vi "HFRR ADV v038.vi"() -> ()   [LabVIEW 2025] (continued)
                    n2637 = local write "Temperature ( Deg C )"(w3212) -> ()
                    n2638 = Number To Fractional String(number=w3190, width (-)=i16 9 ("precision (6)"), precision (6)=i16 6) -> (F-format string=w3236:string)  [unwired: 1 in]
                    n2639 = Number To Fractional String(number=w3216, width (-)=i16 9 ("precision (6)"), precision (6)=i16 3) -> (F-format string=w3235:string)  [unwired: 1 in]
                    n2640 = Number To Fractional String(number=w3212, width (-)=i16 9 ("precision (6)"), precision (6)=i16 3) -> (F-format string=w3232:string)  [unwired: 1 in]
                    n2641 = Number To Fractional String(number=w3211, width (-)=i16 9 ("precision (6)"), precision (6)=i16 3) -> (F-format string=w3229:string)  [unwired: 1 in]
                    n2642 = Number To Fractional String(number=0.0, width (-)=i16 9 ("precision (6)"), precision (6)=i16 3) -> (F-format string=w3226:string)  [unwired: 1 in]
                    n2643 = Number To Fractional String(number=w3221, width (-)=i16 9 ("precision (6)"), precision (6)=i16 3) -> (F-format string=w3222:string)  [unwired: 1 in]
                    n2644 = Number To Fractional String(number=w3218, width (-)=i16 9 ("precision (6)"), precision (6)=i16 3) -> (F-format string=w3217:string)  [unwired: 1 in]
                    n2645 = Number To Fractional String(number=w3209, width (-)=i16 9 ("precision (6)"), precision (6)=i16 6) -> (F-format string=w3244:string)  [unwired: 1 in]
                    n2646 = Number To Fractional String(number=w3243, width (-)=i16 14 ("precision (6)"), precision (6)=i16 3) -> (F-format string=w3245:string)  [unwired: 1 in]
                    n2647 = Bundle("y"=1.02, "LVDT STROKE DISPLAY"=w3190, "y"=0.98) -> (w3210:T31)  [unwired: 1 in]
                    n2648 = Number To Fractional String(number="Ambient Humidity :", width (-)=i16 9 ("precision (6)"), precision (6)=i16 6) -> (F-format string=w3202:string)  [unwired: 1 in]
                    n2649 = local read "RUN"() -> (w3208:bool)
                    n2650 = case shown="True" w3208 {
                      tunnel: w3210 -> [_ w3261]
                      tunnel: w3190 -> [_ w3260]
                      tunnel: w3190 -> [_ w3258]
                      tunnel: w3190 -> [_ w3259]
                      frame False {
                      }
                      frame True {
                        "Stroke ( mm )" <- w3261
                        "Stroke ( mm )" <- w3261
                        "Stroke 4" <- w3260
                        "Stroke 3" <- w3258
                        "Stroke 2" <- w3259
                        "measured_stroke" <- w3258
                      }
                    }
                    n2651 = Concatenate Strings(w3245, w3204, w3244, w3204, w3236, w3204, w3235, w3204, w3232, w3204, w3229, w3204, w3226, w3204, w3222, w3204, w3217, w3204, w3202, "\r") -> (w3242:string)
                    n2652 = call <vilib>:"Write Characters To File.vi"("append to file? (new file:F)"=TRUE, "character string"=w3242, "file path (dialog if empty)"=w3195) -> ()  [unwired: 2 in, 1 out]
                    "refresh flag" <- TRUE ("refresh flag")
                    "LVDT STROKE Actual" <- w3188
                  }
                }
                n2653 = case shown="True" w3110 {
                  tunnel: w3120 -> [_ w3146]
                  tunnel: w3125 -> [_ w3156]
                  tunnel: [0.0 w3152] -> _
                  tunnel: w3119 -> [_ w3151]
                  tunnel: [0.0 w3150] -> _
                  tunnel: w3109 -> [_ w3150]
                  tunnel: w3123 -> [w3139 _]
                  frame False {
                    n2654 = local write "acq timer"(w3139) -> ()
                    n2655 = local write "Test Duration Status"(0.0 ("Test Duration Status")) -> ()
                  }
                  frame True {
                    n2656 = local read "Set Hz"() -> (w3153:dbl)
                    n2657 = local write "Elapsed time"(w3146) -> ()
                    n2658 = local read "test time"() -> (w3145:dbl)
                    n2659 = Multiply(x=w3156, y=w3153) -> (x*y=w3155:dbl)
                    n2660 = case shown="False" w3151 {
                      tunnel: w3155 -> [w3157 _]
                      tunnel: [w3157 1.0] -> w3152
                      frame False {
                        n2661 = local write "Cycles elapsed"(w3157) -> ()
                      }
                      frame True {
                      }
                    }
                    n2662 = Greater?(x=w3146, y=w3145) -> (0:w3154:bool)
                    n2663 = Subtract(x=w3145, y=w3146) -> (x-y=w3144:dbl)
                    n2664 = Multiply(x=w3144, y=60.0) -> (x*y=w3143:dbl)
                    n2665 = local write "Time Remaining"(w3143) -> ()
                    n2666 = local write "Remaining Time"(w3143) -> ()
                    n2667 = case shown="True" w3154 {
                      frame False {
                      }
                      frame True {
                        n2668 = stacked-sequence {
                          frame #0 {
                            w3162 = T19."Enabled" ("Disabled")
                            w3161 = FALSE ("TEST FILE NAM,E SAVED")
                            w3163 = "" ("FILE")
                            w3164 = TRUE ("Visible")
                            n2669 = local write "Humidity"(FALSE ("Humidity")) -> ()
                            n2670 = local write "RUN"(FALSE ("OK Button 2")) -> ()
                            n2671 = local write "Heater Button"(FALSE ("Heater Button")) -> ()
                            n2672 = local write "Auto Start Test"(FALSE ("Auto Start Test")) -> ()
                            n2673 = local write "TestCompFlg"(TRUE ("StpFlg")) -> ()
                            n2674 = local read "Humidity ( %RH )"() -> (→"Rh After":dbl)
                            n2675 = property on="STOP 2" class="Bool (strict)"("Disabled"=u8 0) -> ()  [unwired: 2 in, 2 out]
                            n2676 = local read "EVENT LOG"() -> (w3169:string)
                            n2677 = call "Event Log.vi"("Content"="Test Completed", "EVENT LOG"=w3169) -> ("EVENT LOG"=w3168:string)  [unwired: 8 in, 1 out]
                            n2678 = property on="RUN" class="Bool (strict)"("Visible"=w3164) -> ()  [unwired: 2 in, 2 out]
                            n2679 = property on="Auto Start Test" class="Bool (strict)"("Visible"=w3164) -> ()  [unwired: 2 in, 2 out]
                            n2680 = local write "Batch Ref Num :"(w3163) -> ()
                            n2681 = local write "FILE"(w3163) -> ()
                            n2682 = local write "EVENT LOG"(w3168) -> ()
                            n2683 = local write "TEST FILE NAM,E SAVED"(w3161) -> ()
                            n2684 = local write "Fuel Discription :"(w3163) -> ()
                            n2685 = local write "START TEMP"(w3161) -> ()
                            n2686 = local write "Remarks :"(w3163) -> ()
                            n2687 = local write "Main Dashboard Buttons"(T1."Imaging" ("Main Dashboard Buttons")) -> ()
                            n2688 = local write "Main Tab"(T2."Adv Scar" ("Main Tab")) -> ()
                            n2689 = property on="FRICVALZ 2" class="Bool (strict)"("DisabledEnum"=w3162) -> ()  [unwired: 2 in, 2 out]
                            n2690 = property on="FRICVALZ 3" class="Bool (strict)"("DisabledEnum"=w3162) -> ()  [unwired: 2 in, 2 out]
                            n2691 = property on="FRICVALZ 4" class="Bool (strict)"("DisabledEnum"=w3162) -> ()  [unwired: 2 in, 2 out]
                          }
                          frame #1 {
                            n2692 = Wait (ms)(milliseconds to wait=u32 1500) -> ()  [unwired: 1 out]
                          }
                          frame #2 {
                            n2693 = local write "Due Write"("VC;0") -> ()
                          }
                          frame #3 {
                            n2694 = Wait (ms)(milliseconds to wait=u32 1500) -> ()  [unwired: 1 out]
                          }
                          frame #4 {
                            n2695 = local write "Due Write"("VC;0") -> ()
                          }
                          frame #5 {
                            n2696 = Wait (ms)(milliseconds to wait=u32 1500) -> ()  [unwired: 1 out]
                          }
                          frame #6 {
                            n2697 = local write "Due Write"("ST;0") -> ()
                          }
                          frame #7 {
                            n2698 = local write "measured_stroke"(0.0 ("measured_stroke")) -> ()
                            n2699 = Wait (ms)(milliseconds to wait=u32 1500) -> ()  [unwired: 1 out]
                          }
                          frame #8 {
                            n2700 = local write "Due Write"("HE;0") -> ()
                            n2701 = local write "Humidity"(TRUE ("Humidity")) -> ()
                          }
                        }
                      }
                    }
                    n2702 = Divide(x=w3146, y=w3145) -> (x/y=w3149:dbl)
                    n2703 = Multiply(x=w3149, y=100.0) -> (x*y=w3147:dbl)
                    n2704 = local write "Test Duration Status"(w3147) -> ()
                  }
                }
              }
              frame #2 {
                n2705 = case shown="True" "Heater Button" {
                  tunnel: [0.0 ("output") w3284] -> w3262
                  frame False {
                    w3265 = TRUE ("tmpchk")
                    n2706 = local read "TEMP"() -> (w3266:dbl)
                    n2707 = local write "Temp ini"(w3266) -> ()
                    n2708 = local write "Reset 4"(w3265) -> ()
                    n2709 = local write "tmpchk"(w3265) -> ()
                    n2710 = local write "reinit"(TRUE ("reinit")) -> ()
                    n2711 = local write "manual temp log"(TRUE ("manual temp log")) -> ()
                  }
                  frame True {
                    # "Logic to turn off\nthe heater when \ntemp is not rising.\nTime - 60 sec\nDelta t- 5°c"
                    n2712 = local read "Temp ini"() -> (w3273:dbl)
                    n2713 = local read "Auto Start Test"() -> (w3269:bool)
                    n2714 = Less?(x=w3273, y=53.0) -> (x < y?=w3271:bool)
                    n2715 = case shown="False" w3269 {
                      frame False {
                        n2716 = local read "Set Temp"() -> (w3293:dbl)
                        n2717 = local read "TEMP"() -> (w3292:dbl)
                        n2718 = Subtract(x=w3293, y=w3292) -> (x-y=w3291:dbl)
                        n2719 = Absolute Value(x=w3291) -> (abs(x)=w3290:dbl)
                        n2720 = Less?(x=w3290, y=0.5) -> (x < y?=w3288:bool)
                        n2721 = case shown="True" w3288 {
                          tunnel: "manual temp log" -> [_ w3294]
                          frame False {
                          }
                          frame True {
                            n2722 = case shown="True" w3294 {
                              selector: w3294 -> [_ w3295]
                              frame False {
                              }
                              frame True {
                                # "#Event log"
                                n2723 = Not(x=w3295) -> (.not. x?=w3296:bool)
                                n2724 = local write "manual temp log"(w3296) -> ()
                                n2725 = local read "EVENT LOG"() -> (w3299:string)
                                n2726 = call "Event Log.vi"("Content"="Target Temperature reached", "EVENT LOG"=w3299) -> ("EVENT LOG"=w3298:string)  [unwired: 8 in, 1 out]
                                n2727 = local write "EVENT LOG"(w3298) -> ()
                              }
                            }
                          }
                        }
                      }
                      frame True {
                        n2728 = local write "manual temp log"(TRUE ("manual temp log")) -> ()
                      }
                    }
                    n2729 = And(x="tmpchk", y=w3271) -> (x .and. y?=w3274:bool)
                    n2730 = case shown="True" w3274 {
                      frame False {
                      }
                      frame True {
                        n2731 = call "Elapsed Time8"("Time Target (s)"=300.0, "Reset"="Reset 4") -> ("Time has Elapsed"=w3301:bool)  [unwired: 10 in, 7 out]
                        n2732 = flat-sequence {
                          tunnel: w3301 -> [_]
                          frame #0 {
                            n2733 = local write "Reset 4"(FALSE ("Reset 4")) -> ()
                          }
                        }
                        n2734 = case shown="True" w3301 {
                          frame False {
                          }
                          frame True {
                            n2735 = local read "Temp ini"() -> (w3308:dbl)
                            n2736 = Add(x=w3308, y=5.0) -> (x+y=w3306:dbl)
                            n2737 = local read "TEMP"() -> (w3309:dbl)
                            n2738 = Greater?(x=w3309, y=w3306) -> (0:w3307:bool)
                            n2739 = case shown="False" w3307 {
                              frame False {
                                n2740 = local write "Heater Button"(FALSE ("Heater Button")) -> ()
                              }
                              frame True {
                                n2741 = local write "tmpchk"(FALSE ("tmpchk")) -> ()
                              }
                            }
                          }
                        }
                      }
                    }
                    n2742 = local read "Set Temp"() -> (w3282:dbl)
                    n2743 = local read "TEMP"() -> (w3276:dbl)
                    n2744 = call-poly <vilib>:"PID.vi"("reinitialize? (F)"="reinit", "dt (s)"=-1.0, "process variable"=w3276, "setpoint"=w3282) -> ("output"=w3279:dbl)  [unwired: 6 in, 1 out]
                    n2745 = Subtract(x=w3282, y=w3276) -> (x-y=w3283:dbl)
                    n2746 = Add(x=w3282, y=0.5) -> (x+y=w3280:dbl)
                    n2747 = Greater Or Equal?(x=w3276, y=w3280) -> ()  [unwired: 1 out]
                    n2748 = Select(t=0.0, s=FALSE, f=w3279) -> (s? t:f=w3278:dbl)
                    "PID output" <- w3278
                    n2749 = flat-sequence {
                      tunnel: w3278 -> [w3312]
                      tunnel: [w3312] -> w3284
                      frame #0 {
                        n2750 = local write "reinit"(FALSE ("reinit")) -> ()
                      }
                    }
                    n2751 = Bundle(w3283, "output"=w3278, "TEMP"=w3276) -> ()  [unwired: 1 in, 1 out]
                  }
                }
                "PID-out" <- w3262
              }
              frame #3 {
                n2752 = local read "TEMP"() -> (w3314:dbl)
                n2753 = Greater Or Equal?(x=w3314, y="Set Temp 2") -> (x >= y?=w3319:bool)
                n2754 = case shown="True" w3319 {
                  tunnel: [FALSE TRUE] -> w3317
                  frame False {
                  }
                  frame True {
                  }
                }
                "Status 13" <- w3317
                n2755 = And(x=w3317, y="trip1 8") -> (x .and. y?=w3316:bool)
                n2756 = case shown="True" w3316 {
                  frame False {
                    n2757 = local write "Heater Trip Temp"(TRUE ("Heater Trip Temp")) -> ()
                  }
                  frame True {
                    w3322 = FALSE ("OK Button 2")
                    n2758 = case shown="True" "Heater Trip Temp" {
                      selector: "Heater Trip Temp" -> [_ w3324]
                      frame False {
                      }
                      frame True {
                        n2759 = Not(x=w3324) -> (.not. x?=w3323:bool)
                        n2760 = local read "EVENT LOG"() -> (w3327:string)
                        n2761 = local write "Heater Trip Temp"(w3323) -> ()
                        n2762 = call "Event Log.vi"("Content"="Heater Trip", "EVENT LOG"=w3327) -> ("EVENT LOG"=w3326:string)  [unwired: 8 in, 1 out]
                        n2763 = local write "EVENT LOG"(w3326) -> ()
                      }
                    }
                    n2764 = local write "RUN"(w3322) -> ()
                    n2765 = property on="Auto Start Test" class="Bool (strict)"("Value"=w3322) -> ()  [unwired: 2 in, 2 out]
                    n2766 = local write "Heater Button"(w3322) -> ()
                  }
                }
              }
            }
            n2767 = case shown="False" w3033 {
              frame False {
                n2768 = disable-structure shown="Disabled" {
                  frame Disabled {
                    n2769 = stacked-sequence {
                      frame #0 {
                        n2770 = local write "RUN"(FALSE ("OK Button 2")) -> ()
                      }
                      frame #1 {
                      }
                    }
                  }
                  frame Enabled {
                  }
                }
              }
              frame True {
              }
            }
          }
        }
        n2771 = local read "Reset Graph"() -> (w2930:bool)
        n2772 = case shown="True" w2930 {
          selector: w2930 -> [_ w2947]
          frame False {
          }
          frame True {
            w2961 = 0.0 ("X Scale.Range:Maximum")
            n2773 = Not(x=w2947) -> (.not. x?=w2946:bool)
            n2774 = local write "Reset Graph"(w2946) -> ()
            n2775 = property on="Electrical Contact Resistance ( % )" class="WFChart (strict)"("XScale.Maximum"=600.0 ("X Scale.Range:Maximum"), "XScale.Minimum"=0.0 ("X Scale.Range:Minimum"), "YScale.Maximum"=100.0 ("Y Scale.Range:Maximum"), "YScale.Minimum"=0.0 ("Y Scale.Range:Minimum")) -> ()  [unwired: 2 in, 2 out]
            n2776 = property on="Frictional Force ( N )" class="WFChart (strict)"("XScale.Maximum"=600.0 ("X Scale.Range:Maximum"), "XScale.Minimum"=0.0 ("X Scale.Range:Minimum"), "YScale.Maximum"=100.0 ("Y Scale.Range:Maximum"), "YScale.Minimum"=0.0 ("Y Scale.Range:Minimum")) -> ()  [unwired: 2 in, 2 out]
            n2777 = property on="Temperature ( Deg C )" class="WFChart (strict)"("XScale.Maximum"=600.0 ("X Scale.Range:Maximum"), "XScale.Minimum"=0.0 ("X Scale.Range:Minimum"), "YScale.Maximum"=100.0 ("Y Scale.Range:Maximum"), "YScale.Minimum"=0.0 ("Y Scale.Range:Minimum")) -> ()  [unwired: 2 in, 2 out]
            n2778 = property on="Stroke ( mm )" class="WFChart (strict)"("XScale.Maximum"=600.0 ("X Scale.Range:Maximum"), "XScale.Minimum"=0.0 ("X Scale.Range:Minimum"), "YScale.Maximum"=100.0 ("Y Scale.Range:Maximum"), "YScale.Minimum"=0.0 ("Y Scale.Range:Minimum")) -> ()  [unwired: 2 in, 2 out]
            n2779 = property on="Coefficient of Friction" class="WFChart (strict)"("XScale.Maximum"=600.0 ("X Scale.Range:Maximum"), "XScale.Minimum"=0.0 ("X Scale.Range:Minimum"), "YScale.Maximum"=100.0 ("Y Scale.Range:Maximum"), "YScale.Minimum"=0.0 ("Y Scale.Range:Minimum")) -> ()  [unwired: 2 in, 2 out]
            n2780 = property on="Electrical Contact Resistance ( % )" class="WFChart (strict)"("XScale.Minimum"=0.0 ("X Scale.Range:Minimum"), "XScale.Maximum"=600.0 ("X Scale.Range:Maximum"), "YScale.Minimum"=0.0 ("Y Scale.Range:Minimum"), "YScale.Maximum"=100.0 ("Y Scale.Range:Maximum")) -> ()  [unwired: 2 in, 2 out]
            n2781 = property on="Temperature ( Deg C )" class="WFChart (strict)"("XScale.Minimum"=0.0 ("X Scale.Range:Minimum"), "XScale.Maximum"=600.0 ("X Scale.Range:Maximum"), "YScale.Minimum"=0.0 ("Y Scale.Range:Minimum"), "YScale.Maximum"=100.0 ("Y Scale.Range:Maximum")) -> ()  [unwired: 2 in, 2 out]
            n2782 = property on="Coefficient of Friction" class="WFChart (strict)"("XScale.Minimum"=0.0 ("X Scale.Range:Minimum"), "XScale.Maximum"=600.0 ("X Scale.Range:Maximum"), "YScale.Maximum"=1.0 ("X Scale.Range:Minimum"), "YScale.Minimum"=0.0 ("X Scale.Range:Minimum")) -> ()  [unwired: 2 in, 2 out]
            n2783 = property on="Frictional Force ( N )" class="WFChart (strict)"("XScale.Maximum"=600.0 ("X Scale.Range:Maximum"), "XScale.Minimum"=w2961, "YScale.Maximum"=10.0 ("Y Scale.Range:Maximum"), "YScale.Minimum"=w2961) -> ()  [unwired: 2 in, 2 out]
            n2784 = property on="Stroke ( mm )" class="WFChart (strict)"("XScale.Maximum"=600.0 ("X Scale.Range:Maximum"), "XScale.Minimum"=0.0 ("X Scale.Range:Minimum"), "YScale.Maximum"=100.0 ("Y Scale.Range:Maximum"), "YScale.Minimum"=0.0 ("Y Scale.Range:Minimum")) -> ()  [unwired: 2 in, 2 out]
          }
        }
      }
      frame "Compare Files" {
        # "Elapsed time\ncof\nstroke\nAir temp\nTemp\nHumidity"
        n2785 = case shown="True" "RSTV1 2" {
          frame False {
          }
          frame True {
            n2786 = property on="Humidity ( %RH )" class="XYGraph (strict)"("Y Scale.Display Format:Precision"=u8 0 ("Y Scale.Format & Precision:Precision")) -> ()  [unwired: 2 in, 2 out]
            n2787 = property on="Humidity ( %RH )" class="XYGraph (strict)"("X Scale.Range:Minimum"=0.0, "X Scale.Range:Maximum"=75.0, "Y Scale.Range:Minimum"=48.0, "Y Scale.Range:Maximum"=58.0) -> ()  [unwired: 2 in, 2 out]
          }
        }
        n2788 = case shown="True" "RST CP 2" {
          frame False {
          }
          frame True {
            n2789 = property on="XY Graph 13" class="XYGraph (strict)"("Y Scale.Display Format:Precision"=u8 0 ("Y Scale.Format & Precision:Precision")) -> ()  [unwired: 2 in, 2 out]
            n2790 = property on="XY Graph 13" class="XYGraph (strict)"("X Scale.Range:Minimum"=0.0, "X Scale.Range:Maximum"=75.0, "Y Scale.Range:Minimum"=0.0, "Y Scale.Range:Maximum"=100.0) -> ()  [unwired: 2 in, 2 out]
          }
        }
        n2791 = case shown="True" "RST CP" {
          frame False {
          }
          frame True {
            n2792 = property on="Sample Temperature ( °C )" class="XYGraph (strict)"("Y Scale.Display Format:Precision"=u8 2 ("Y Scale.Format & Precision:Precision")) -> ()  [unwired: 2 in, 2 out]
            n2793 = property on="Sample Temperature ( °C )" class="XYGraph (strict)"("X Scale.Range:Minimum"=0.0, "X Scale.Range:Maximum"=75.0, "Y Scale.Range:Minimum"=58.0, "Y Scale.Range:Maximum"=62.0) -> ()  [unwired: 2 in, 2 out]
          }
        }
        n2794 = case shown="True" "RSTV1 3" {
          frame False {
          }
          frame True {
            n2795 = property on="Air Temperature  ( °C )" class="XYGraph (strict)"("Y Scale.Display Format:Precision"=u8 2 ("Y Scale.Format & Precision:Precision")) -> ()  [unwired: 2 in, 2 out]
            n2796 = property on="Air Temperature  ( °C )" class="XYGraph (strict)"("X Scale.Range:Minimum"=0.0 ("Y Scale.Range:Minimum"), "X Scale.Range:Maximum"=75.0 ("Y Scale.Range:Maximum"), "Y Scale.Range:Minimum"=20.0 ("X Scale.Range:Minimum"), "Y Scale.Range:Maximum"=26.0 ("X Scale.Range:Maximum")) -> ()  [unwired: 2 in, 2 out]
          }
        }
        n2797 = case shown="True" "RSTV1 4" {
          frame False {
          }
          frame True {
            n2798 = property on="Stroke ( mm )" class="XYGraph (strict)"("Y Scale.Display Format:Precision"=u8 2 ("Y Scale.Format & Precision:Precision")) -> ()  [unwired: 2 in, 2 out]
            n2799 = property on="Stroke ( mm )" class="XYGraph (strict)"("X Scale.Range:Minimum"=0.0 ("Y Scale.Range:Maximum"), "X Scale.Range:Maximum"=75.0 ("X Scale.Range:Minimum"), "Y Scale.Range:Minimum"=0.98, "Y Scale.Range:Maximum"=1.02) -> ()  [unwired: 2 in, 2 out]
          }
        }
        n2800 = case shown="True" "rstv2" {
          frame False {
          }
          frame True {
            n2801 = property on="Coefficient Of Friction" class="XYGraph (strict)"("Y Scale.Display Format:Precision"=u8 3 ("Y Scale.Format & Precision:Precision")) -> ()  [unwired: 2 in, 2 out]
            n2802 = property on="Coefficient Of Friction" class="XYGraph (strict)"("X Scale.Range:Minimum"=0.0 ("Y Scale.Range:Maximum"), "X Scale.Range:Maximum"=75.0, "Y Scale.Range:Minimum"=0.0, "Y Scale.Range:Maximum"=1.0 ("X Scale.Range:Minimum")) -> ()  [unwired: 2 in, 2 out]
          }
        }
        n2803 = case shown="True" "RST CP 3" {
          frame False {
          }
          frame True {
            n2804 = property on="Air Temp ( °C ) vs Humidity ( % RH )" class="XYGraph (strict)"("X Scale.Range:Minimum"=18.0, "X Scale.Range:Maximum"=28.0 ("X Scale.Range:Minimum"), "Y Scale.Range:Minimum"=30.0 ("X Scale.Range:Minimum"), "Y Scale.Range:Maximum"=70.0 ("X Scale.Range:Minimum")) -> ()  [unwired: 2 in, 2 out]
          }
        }
        n2805 = case shown="True" "OPEN 1" {
          frame False {
          }
          frame True {
            (unwired) 0  # existing file
            w3603 = "Choose a datalog file to open"  # prompt
            n2806 = local write "OPEN 1"(FALSE ("OPEN 1")) -> ()
            n2807 = String To Path(string="C:\\LAB-IQ\\Data\\") -> (path=w3588:path)
            n2808 = File Dialog(6:"*.dgf" ("pattern"), 7:w3603, 11:w3588) -> (0:w3586:errorcluster, 3:w3594:path)  [unwired: 4 in, 2 out]
            n2809 = Unbundle(w3586) -> ()  [unwired: 3 out]
            n2810 = Strip Path(path=w3594) -> (name=w3593:string)  [unwired: 1 out]
            n2811 = Path To String(path=w3594) -> (string=w3589:string)
            "string1" <- w3589
            n2812 = Match Pattern(string=w3593, regular expression=".dgf") -> (before substring=→"String Control":string)  [unwired: 1 in, 3 out]
            n2813 = Match Pattern(string=w3589, regular expression=".dgf" ("substring (\"\")")) -> (before substring=w3599:string)  [unwired: 1 in, 3 out]
            n2814 = Concatenate Strings(w3599, ".duf" ("Substring")) -> (w3595:string)
            n2815 = String To Path(string=w3595) -> (path=w3600:path)
            n2816 = call <vilib>:"Read Characters From File.vi"("file path (dialog if empty)"=w3600, "start of read offset (chars.:0)"=60 ("start of read offset (chars.: 0)")) -> ("character string"=→"String Control 2":string)  [unwired: 4 in, 3 out]
          }
        }
        n2817 = case shown="True" "OPEN 2" {
          frame False {
          }
          frame True {
            (unwired) 0  # existing file
            w3621 = "Choose a datalog file to open"  # prompt
            n2818 = local write "OPEN 2"(FALSE ("OPEN 1")) -> ()
            n2819 = String To Path(string="C:\\LAB-IQ\\Data\\") -> (path=w3606:path)
            n2820 = File Dialog(6:"*.dgf" ("pattern"), 7:w3621, 11:w3606) -> (0:w3604:errorcluster, 3:w3612:path)  [unwired: 4 in, 2 out]
            n2821 = Unbundle(w3604) -> ()  [unwired: 3 out]
            n2822 = Strip Path(path=w3612) -> (name=w3610:string)  [unwired: 1 out]
            n2823 = Path To String(path=w3612) -> (string=w3607:string)
            "string1 2" <- w3607
            n2824 = Match Pattern(string=w3610, regular expression=".dgf") -> (before substring=→"String Control 3":string)  [unwired: 1 in, 3 out]
            n2825 = Match Pattern(string=w3607, regular expression=".dgf" ("substring (\"\")")) -> (before substring=w3618:string)  [unwired: 1 in, 3 out]
            n2826 = Concatenate Strings(w3618, ".duf" ("Substring")) -> (w3615:string)
            n2827 = String To Path(string=w3615) -> (path=w3613:path)
            n2828 = call <vilib>:"Read Characters From File.vi"("file path (dialog if empty)"=w3613, "start of read offset (chars.:0)"=60 ("start of read offset (chars.: 0)")) -> ("character string"=→"String Control 4":string)  [unwired: 4 in, 3 out]
          }
        }
        n2829 = case shown="True" "OPEN 3" {
          frame False {
          }
          frame True {
            (unwired) 0  # existing file
            w3639 = "Choose a datalog file to open"  # prompt
            n2830 = local write "OPEN 3"(FALSE ("OPEN 1")) -> ()
            n2831 = String To Path(string="C:\\LAB-IQ\\Data\\") -> (path=w3624:path)
            n2832 = File Dialog(6:"*.dgf" ("pattern"), 7:w3639, 11:w3624) -> (0:w3622:errorcluster, 3:w3630:path)  [unwired: 4 in, 2 out]
            n2833 = Unbundle(w3622) -> ()  [unwired: 3 out]
            n2834 = Strip Path(path=w3630) -> (name=w3628:string)  [unwired: 1 out]
            n2835 = Path To String(path=w3630) -> (string=w3625:string)
            "string1 3" <- w3625
            n2836 = Match Pattern(string=w3628, regular expression=".dgf") -> (before substring=→"String Control 5":string)  [unwired: 1 in, 3 out]
            n2837 = Match Pattern(string=w3625, regular expression=".dgf" ("substring (\"\")")) -> (before substring=w3635:string)  [unwired: 1 in, 3 out]
            n2838 = Concatenate Strings(w3635, ".duf" ("Substring")) -> (w3632:string)
            n2839 = String To Path(string=w3632) -> (path=w3636:path)
            n2840 = call <vilib>:"Read Characters From File.vi"("file path (dialog if empty)"=w3636, "start of read offset (chars.:0)"=60 ("start of read offset (chars.: 0)")) -> ("character string"=→"String Control 6":string)  [unwired: 4 in, 3 out]
          }
        }
        n2841 = case shown="True" "OPEN 4" {
          frame False {
          }
          frame True {
            (unwired) 0  # existing file
            w3657 = "Choose a datalog file to open"  # prompt
            n2842 = local write "OPEN 4"(FALSE ("OPEN 1")) -> ()
            n2843 = String To Path(string="C:\\LAB-IQ\\Data\\") -> (path=w3642:path)
            n2844 = File Dialog(6:"*.dgf" ("pattern"), 7:w3657, 11:w3642) -> (0:w3640:errorcluster, 3:w3648:path)  [unwired: 4 in, 2 out]
            n2845 = Unbundle(w3640) -> ()  [unwired: 3 out]
            n2846 = Strip Path(path=w3648) -> (name=w3646:string)  [unwired: 1 out]
            n2847 = Path To String(path=w3648) -> (string=w3643:string)
            "string1 4" <- w3643
            n2848 = Match Pattern(string=w3646, regular expression=".dgf") -> (before substring=→"String Control 7":string)  [unwired: 1 in, 3 out]
            n2849 = Match Pattern(string=w3643, regular expression=".dgf" ("substring (\"\")")) -> (before substring=w3653:string)  [unwired: 1 in, 3 out]
            n2850 = Concatenate Strings(w3653, ".duf" ("Substring")) -> (w3650:string)
            n2851 = String To Path(string=w3650) -> (path=w3654:path)
            n2852 = call <vilib>:"Read Characters From File.vi"("file path (dialog if empty)"=w3654, "start of read offset (chars.:0)"=60 ("start of read offset (chars.: 0)")) -> ("character string"=→"String Control 8":string)  [unwired: 4 in, 3 out]
          }
        }
      }
      frame "About" {
        # "Elapsed time\ncof\nstroke\nmean pos\nTemp\nHumidity"
        n2853 = disable-structure shown="Disabled" {
          frame Disabled {
            n2854 = case shown="True" "Export" {
              frame False {
              }
              frame True {
                w3679 = "                                      " ("string")
                w3681 = "\r"
                (unwired) i16 6 ("width (-)")
                w3758 = "\r"
                w3690 = "\r"
                n2855 = local write "Export"(FALSE ("Export")) -> ()
                n2856 = local read "String 29"() -> (w3727:string)
                n2857 = local read "String 34"() -> (w3715:string)
                n2858 = local read "String 35"() -> (w3710:string)
                n2859 = local read "String 37"() -> (w3706:string)
                n2860 = local read "String 36"() -> (w3703:string)
                n2861 = local read "String 38"() -> (w3700:string)
                n2862 = local read "String 39"() -> (w3697:string)
                n2863 = Match Pattern(string=w3727, regular expression=".dwm") -> (before substring=w3723:string)  [unwired: 1 in, 3 out]
                "before substring" <- w3723
                n2864 = local read "S 38"() -> (w3718:string)
                n2865 = local read "S 39"() -> (w3711:string)
                n2866 = local read "Temperature before test 2"() -> (w3747:dbl)
                n2867 = local read "Temperature after test 2"() -> (w3752:dbl)
                n2868 = local read "Humidity before test 2"() -> (w3733:dbl)
                n2869 = local read "Humidity after test 2"() -> (w3748:dbl)
                n2870 = local read "MWSD 2"() -> (w3744:dbl)
                n2871 = local read "WS1.4 2"() -> (w3760:dbl)
                n2872 = local read "HCF 2"() -> (w3756:dbl)
                n2873 = local read "AVP 2"() -> (w3745:dbl)
                n2874 = Concatenate Strings("1," ("string"), w3718) -> (w3717:string)
                n2875 = Concatenate Strings("2," ("string"), w3715) -> (w3714:string)
                n2876 = Concatenate Strings("3," ("string"), w3711) -> (w3713:string)
                n2877 = Concatenate Strings("4," ("string"), w3710) -> (w3709:string)
                n2878 = Concatenate Strings("5," ("string"), w3706) -> (w3707:string)
                n2879 = Concatenate Strings("6," ("string"), w3703) -> (w3704:string)
                n2880 = Concatenate Strings("7," ("string"), w3700) -> (w3701:string)
                n2881 = Concatenate Strings("8," ("string"), w3697) -> (w3698:string)
                n2882 = local read "Sample ID"() -> (w3765:string)
                n2883 = case shown="\"xlx\"" "Select File Type" {
                  tunnel: w3723 -> [w3768 w3770 w3772]
                  tunnel: [w3766 w3771 w3773] -> w3722
                  frame "xlx" {
                    n2884 = Concatenate Strings(w3768, ".xls" ("string")) -> (w3766:string)
                  }
                  frame "csv" {
                    n2885 = Concatenate Strings(w3770, ".csv" ("string")) -> (w3771:string)
                  }
                  frame "txt" {
                    n2886 = Concatenate Strings(w3772, ".txt" ("string")) -> (w3773:string)
                  }
                }
                n2887 = local read "Test Date"() -> (w3764:string)
                n2888 = local read "String 45"() -> (w3678:string)
                n2889 = local read "String 31"() -> (w3763:string)
                n2890 = local read "String 32"() -> (w3762:string)
                n2891 = local read "TITTLE"() -> (w3686:string)
                n2892 = Number To Fractional String(number=w3733, width (-)=i16 6, precision (6)=i16 2) -> (F-format string=w3732:string)  [unwired: 1 in]
                n2893 = Number To Fractional String(number=w3747, width (-)=i16 6, precision (6)=i16 2) -> (F-format string=w3753:string)  [unwired: 1 in]
                n2894 = Number To Fractional String(number=w3748, width (-)=i16 6, precision (6)=i16 2) -> (F-format string=w3746:string)  [unwired: 1 in]
                n2895 = Number To Fractional String(number=w3752, width (-)=i16 6, precision (6)=i16 2) -> (F-format string=w3751:string)  [unwired: 1 in]
                n2896 = Number To Fractional String(number=w3744, width (-)=i16 6, precision (6)=i16 2) -> (F-format string=w3742:string)  [unwired: 1 in]
                n2897 = Number To Fractional String(number=w3745, width (-)=i16 6, precision (6)=i16 2) -> (F-format string=w3743:string)  [unwired: 1 in]
                n2898 = Number To Fractional String(number=w3756, width (-)=i16 6, precision (6)=i16 2) -> (F-format string=w3757:string)  [unwired: 1 in]
                n2899 = Number To Fractional String(number=w3760, precision (6)=i16 2) -> (F-format string=w3761:string)  [unwired: 2 in]
                n2900 = local read "s.NO"() -> (w3680:string)
                n2901 = Concatenate Strings("=" ("string"), w3686) -> (w3685:string)
                n2902 = Concatenate Strings("S.No," ("string"), "                                       Parameters" ("string")) -> (w3691:string)
                n2903 = Concatenate Strings(w3758, w3717, w3732, w3758, w3714, w3753, w3758, w3713, w3746, w3758, w3709, w3751, w3758, w3707, w3742, w3758, w3704, w3743, w3758, w3701, w3757, w3758, w3698, w3761) -> (w3720:string)
                n2904 = Concatenate Strings(w3690, "," ("string"), w3678, w3680, w3679, w3762, w3765, w3679, w3763, w3764, w3690) -> (w3688:string)
                n2905 = local read "Tested by"() -> (w3694:string)
                n2906 = local read "String 33"() -> (w3695:string)
                n2907 = Concatenate Strings("," ("string"), "                                                                             " ("string")) -> (w3683:string)
                n2908 = Concatenate Strings(w3685, w3681, w3688, w3681, w3691, w3720, w3681, w3683, w3695, w3694) -> (→"export":string)
                n2909 = String To Path(string=w3722) -> (path=w3729:path)
                n2910 = local read "export"() -> (w3724:string)
                n2911 = call <vilib>:"Write Characters To File.vi"("append to file? (new file:F)"=FALSE, "character string"=w3724, "file path (dialog if empty)"=w3729) -> ()  [unwired: 2 in, 1 out]
              }
            }
          }
          frame Enabled {
          }
        }
        n2912 = case shown="True" "OK Button 17" {
          frame False {
          }
          frame True {
            (unwired) 0  # existing file
            w3982 = "Choose a datalog file to open"  # prompt
            n2913 = local write "OK Button 17"(FALSE ("OK Button 17")) -> ()
            n2914 = local read "String"() -> (w3977:string)
            n2915 = String To Path(string=w3977) -> (path=w3978:path)
            n2916 = File Dialog(6:"*.duf" ("pattern"), 7:w3982, 11:w3978) -> (0:w3969:errorcluster, 3:w3988:path)  [unwired: 4 in, 2 out]
            n2917 = Unbundle(w3969) -> ()  [unwired: 3 out]
            n2918 = Open/Create/Replace File "Open File"(file path (use dialog)=w3988) -> (refnum out=w3980:refnum<file>)  [unwired: 5 in, 2 out]
            n2919 = Strip Path(path=w3988) -> (name=w3986:string)  [unwired: 1 out]
            n2920 = Path To String(path=w3988) -> (string=w3971:string)
            n2921 = while {
              tunnel: w3980 -> [w3992]
              i -> [w3989]
              stop <- w3990 continue-if-true
              (unwired) TRUE ("line mode (F)")
              n2922 = Read from Text File "Read File"(file (use dialog)=w3992) -> (text=w3991:string)  [unwired: 3 in, 3 out]
              n2923 = local write "Numeric 16"(w3989) -> ()
              n2924 = String Length(string=w3991) -> (length=w3994:i32)
              n2925 = Greater?(x=w3994, y=1) -> (0:w3990:bool)
            }
            n2926 = local write "String 29"(w3971) -> ()
            n2927 = Search and Replace String(input string=w3971, search string=".duf", replace string=".dgf" ("replace string (\"\")")) -> (result string=→"String Indicator 4":string)  [unwired: 5 in, 3 out]
            n2928 = Match Pattern(string=w3986, regular expression=".dwm") -> (before substring=w3970:string)  [unwired: 1 in, 3 out]
            "String Indicator" <- w3970
            n2929 = Match Pattern(string=w3971, regular expression=".dwm" ("substring (\"\")")) -> (before substring=w3972:string)  [unwired: 1 in, 3 out]
            "String Indicator 3" <- w3972
            n2930 = local write "TITTLE 2"(w3970) -> ()
            n2931 = String To Path(string=w3972) -> (path=w3979:path)
            "path" <- w3979
            n2932 = call <vilib>:"Read Characters From File.vi"("file path (dialog if empty)"=w3979, "start of read offset (chars.:0)"=60 ("start of read offset (chars.: 0)")) -> ("character string"=→"String Indicator 2":string)  [unwired: 4 in, 3 out]
          }
        }
        n2933 = call <vilib>:"Query Available Printers.vi"() -> ("system configured printers"=w3671:string[])  [unwired: 9 in, 2 out]
        "System Configured Printers 2" <- w3671
        n2934 = local read "OK Button 16"() -> (w3668:bool)
        n2935 = case shown="True" "OK Button 16" {
          frame False {
          }
          frame True {
            n2936 = stacked-sequence {
              frame #0 {
                n2937 = local read "Numeric 16"() -> (w3996:i32)
                n2938 = local write "Numeric 10"(w3996) -> ()
              }
              frame #1 {
                n2939 = local read "String 29"() -> (w3999:string)
                n2940 = String To Path(string=w3999) -> (path=w3998:path)
                n2941 = Open/Create/Replace File "Open File"(file path (use dialog)=w3998) -> (refnum out=w4000:refnum<file>)  [unwired: 5 in, 2 out]
                n2942 = for {
                  N: 16 -> [_]
                  tunnel: w4000 -> [w4007]
                  i -> [w4003]
                  (unwired) TRUE ("line mode (F)")
                  n2943 = Read from Text File "Read File"(file (use dialog)=w4007) -> (text=w4001:string)  [unwired: 3 in, 3 out]
                  n2944 = Match Pattern(string=w4001, regular expression="(") -> (after substring=w4006:string)  [unwired: 1 in, 3 out]
                  n2945 = Match Pattern(string=w4006, regular expression=")") -> (before substring=w4002:string)  [unwired: 1 in, 3 out]
                  n2946 = case shown="1" w4003 {
                    tunnel: w4002 -> [w4008 w4009 _ _ w4010 w4011 w4012 w4014 w4016 w4018 w4020 w4022 w4024 w4026 _]
                    tunnel: w4001 -> [_ _ _ _ _ _ _ _ _ _ _ _ _ _ _]
                    frame 0 {
                      "TITTLE" <- w4008
                    }
                    frame 1 {
                      "Sample ID" <- w4009
                    }
                    frame 2 {
                    }
                    frame 3 {
                    }
                    frame 4 {
                      "Test Date" <- w4010
                    }
                    frame 5 {
                      "Tested by" <- w4011
                    }
                    frame 6 {
                      n2947 = Fract/Exp String To Number(string=w4012) -> (number=→"Humidity before test 2":dbl)  [unwired: 3 in, 1 out]
                    }
                    frame 7 {
                      n2948 = Fract/Exp String To Number(string=w4014) -> (number=→"Temperature before test 2":dbl)  [unwired: 3 in, 1 out]
                    }
                    frame 8 {
                      n2949 = Fract/Exp String To Number(string=w4016) -> (number=→"Humidity after test 2":dbl)  [unwired: 3 in, 1 out]
                    }
                    frame 9 {
                      n2950 = Fract/Exp String To Number(string=w4018) -> (number=→"Temperature after test 2":dbl)  [unwired: 3 in, 1 out]
                    }
                    frame 10 {
                      n2951 = Fract/Exp String To Number(string=w4020) -> (number=→"MWSD 2":dbl)  [unwired: 3 in, 1 out]
                    }
                    frame 11 {
                      n2952 = Fract/Exp String To Number(string=w4022) -> (number=→"AVP 2":dbl)  [unwired: 3 in, 1 out]
                    }
                    frame 12 {
                      n2953 = Fract/Exp String To Number(string=w4024) -> (number=→"HCF 2":dbl)  [unwired: 3 in, 1 out]
                    }
                    frame 13 {
                      n2954 = Fract/Exp String To Number(string=w4026) -> (number=→"WS1.4 2":dbl)  [unwired: 3 in, 1 out]
                    }
                    frame 14, Default {
                    }
                  }
                }
              }
              frame #2 {
              }
            }
            n2955 = local write "OK Button 16"(FALSE ("OK Button 13")) -> ()
          }
        }
        n2956 = Index Array(array=w3671, index="Select Printer 3") -> (element=w3673:string)
        "Selected Printer" <- w3673
        n2957 = case shown="True" w3668 {
          frame False {
          }
          frame True {
            n2958 = flat-sequence {
              frame #0 {
              }
              frame #1 {
                n2959 = Wait (ms)(milliseconds to wait=u32 100) -> ()  [unwired: 1 out]
              }
              frame #2 {
                n2960 = local write "OK Button 16"(FALSE ("Print 3")) -> ()
              }
            }
          }
        }
        n2961 = case shown="True" "Print" {
          tunnel: w3673 -> [_ w3965]
          frame False {
          }
          frame True {
            (unwired) i16 6 ("width (-)")
            (unwired) "TESTED BY : "
            (unwired) "TESTED DATE :"
            (unwired) "SAMPLE ID : "
            (unwired) "SAMPLE DESIGN : "
            w3923 = "\r"
            w3940 = "\r"
            # "add image"
            n2962 = local read "Sample ID"() -> (w3913:string)
            n2963 = local read "Tested by"() -> (w3916:string)
            n2964 = local read "String 34"() -> (w3903:string)
            n2965 = local read "String 45"() -> (w3883:string)
            n2966 = local read "String 35"() -> (w3898:string)
            n2967 = local read "String 37"() -> (w3896:string)
            n2968 = local read "String 32"() -> (w3918:string)
            n2969 = local read "String 36"() -> (w3893:string)
            n2970 = local read "String 31"() -> (w3917:string)
            n2971 = local read "Test Date"() -> (w3914:string)
            n2972 = local read "String 33"() -> (w3919:string)
            n2973 = local read "String 38"() -> (w3889:string)
            n2974 = local read "String 39"() -> (w3886:string)
            n2975 = local write "Print"(FALSE ("Print FF")) -> ()
            n2976 = local read "S 39"() -> (w3901:string)
            n2977 = local read "S 38"() -> (w3908:string)
            n2978 = local read "Temperature before test 2"() -> (w3939:dbl)
            n2979 = local read "Temperature after test 2"() -> (w3929:dbl)
            n2980 = local read "Humidity before test 2"() -> (w3954:dbl)
            n2981 = local read "Humidity after test 2"() -> (w3938:dbl)
            n2982 = local read "MWSD 2"() -> (w3943:dbl)
            n2983 = local read "WS1.4 2"() -> (w3921:dbl)
            n2984 = Concatenate Strings("2)" ("string"), w3903) -> (w3904:string)
            n2985 = Concatenate Strings("3)" ("string"), w3901) -> (w3902:string)
            n2986 = Concatenate Strings("1)" ("string"), w3908) -> (w3907:string)
            n2987 = Concatenate Strings("4)" ("string"), w3898) -> (w3899:string)
            n2988 = Concatenate Strings("5)" ("string"), w3896) -> (w3895:string)
            n2989 = Concatenate Strings("6)" ("string"), w3893) -> (w3892:string)
            n2990 = Concatenate Strings("7)" ("string"), w3889) -> (w3890:string)
            n2991 = Concatenate Strings("8)" ("string"), w3886) -> (w3887:string)
            n2992 = local read "HCF 2"() -> (w3925:dbl)
            n2993 = local read "AVP 2"() -> (w3942:dbl)
            n2994 = local read "s.NO"() -> (w3884:string)
            n2995 = call <vilib>:"New Report.vi"("report type"=enum16{"Standard Report", "HTML"}."Standard Report") -> ("report out"=w3963:refnum<class "NI_report.lvclass">, "error out"=w3962:errorcluster)  [unwired: 13 in]
            n2996 = local read "TITTLE"() -> (w3915:string)
            n2997 = Concatenate Strings(w3940, w3883, w3884, w3940, w3918, w3913, w3940, w3917, w3914, w3940, w3919, w3916, w3940) -> (w3933:string)
            "test by" <- w3933
            n2998 = Number To Fractional String(number=w3939, width (-)=i16 6, precision (6)=i16 2) -> (F-format string=w3928:string)  [unwired: 1 in]
            n2999 = Number To Fractional String(number=w3938, width (-)=i16 6, precision (6)=i16 2) -> (F-format string=w3941:string)  [unwired: 1 in]
            n3000 = Number To Fractional String(number=w3954, width (-)=i16 6, precision (6)=i16 2) -> (F-format string=w3959:string)  [unwired: 1 in]
            n3001 = Number To Fractional String(number=w3943, width (-)=i16 6, precision (6)=i16 2) -> (F-format string=w3945:string)  [unwired: 1 in]
            n3002 = Number To Fractional String(number=w3929, width (-)=i16 6, precision (6)=i16 2) -> (F-format string=w3930:string)  [unwired: 1 in]
            n3003 = Number To Fractional String(number=w3942, width (-)=i16 6, precision (6)=i16 2) -> (F-format string=w3944:string)  [unwired: 1 in]
            n3004 = Number To Fractional String(number=w3925, width (-)=i16 6, precision (6)=i16 2) -> (F-format string=w3924:string)  [unwired: 1 in]
            n3005 = Number To Fractional String(number=w3921, precision (6)=i16 2) -> (F-format string=w3920:string)  [unwired: 2 in]
            n3006 = call-dynamic "Set Report Header Text.vi"("report in"=w3963, "center header text"=w3915, "error in (no error)"=w3962) -> ("report out"=w3934:refnum<class "NI_report.lvclass">, "error out"=w3935:errorcluster)  [unwired: 11 in]
            n3007 = Concatenate Strings(w3923, w3907, w3959, w3923, w3904, w3928, w3923, w3902, w3941, w3923, w3899, w3930, w3923, w3895, w3945, w3923, w3892, w3944, w3923, w3890, w3924, w3923, w3887, w3920) -> (w3911:string)
            "export 2" <- w3911
            n3008 = call-poly <vilib>:"Append Report Text.vi"("report in"=w3934, "text"=w3933, "error in (no error)"=w3935) -> ("report out"=w3937:refnum<class "NI_report.lvclass">, "error out"=w3936:errorcluster)  [unwired: 9 in, 2 out]
            n3009 = local read "test by"() -> (w3910:string)
            n3010 = local read "TITTLE"() -> (w3912:string)
            n3011 = call-poly <vilib>:"Append Report Text.vi"("report in"=w3937, "error in (no error)"=w3936) -> ("report out"=w3958:refnum<class "NI_report.lvclass">, "error out"=w3956:errorcluster)  [unwired: 10 in, 2 out]
            n3012 = Concatenate Strings(w3912, w3911, w3910) -> (→"output":string)
            n3013 = call-poly <vilib>:"Append Report Text.vi"("report in"=w3958, "text"=w3911, "error in (no error)"=w3956) -> ("report out"=w3957:refnum<class "NI_report.lvclass">, "error out"=w3955:errorcluster)  [unwired: 9 in, 2 out]
            n3014 = call-dynamic "Print Report.vi"("report in"=w3957, "printer name (default)"=w3965, "error in (no error)"=w3955) -> ("report out"=w3967:refnum<class "NI_report.lvclass">, "error out"=w3968:errorcluster)  [unwired: 11 in]
            n3015 = call-dynamic "Dispose Report.vi"("report in"=w3967, "error in (no error)"=w3968) -> ()  [unwired: 13 in, 1 out]
          }
        }
        n3016 = case shown="True" "Print 2" {
          frame False {
          }
          frame True {
            n3017 = flat-sequence {
              frame #0 {
                n3018 = local read "s.NO"() -> (→"s.NO 2":string)
                n3019 = Wait (ms)(milliseconds to wait=u32 20) -> ()  [unwired: 1 out]
                n3020 = local read "Sample ID  3"() -> (→"Sample ID  6":string)
                n3021 = local read "Sample ID  4"() -> (→"Sample ID  7":string)
                n3022 = local read "Sample ID"() -> (→"Sample ID  2":string)
                n3023 = local read "Tested by"() -> (→"Tested by 2":string)
                n3024 = local read "Test Date"() -> (→"Test Date 2":string)
                n3025 = local read "Humidity after test 3"() -> (→"Humidity after test 4":dbl)
                n3026 = local read "Ref A Test Date :"() -> (→"TITTLE 4":string)
                n3027 = local read "Temperature before test 3"() -> (w3790:dbl)
                n3028 = local read "Temperature before test 3"() -> (→"Temperature after test 5":dbl)
                n3029 = local read "Temperature after test 3"() -> (→"Temperature after test 4":dbl)
                n3030 = local read "Humidity before test 3"() -> (→"Humidity before test 4":dbl)
                n3031 = local write "Temperature before test 3"(w3790) -> ()
                n3032 = local read "image data"() -> (w3781:T16)
                n3033 = String To Path(string="C:\\LAB-IQ\\im\\Temp_resized.jpg") -> (path=w3782:path)
                "path 2" <- w3782
                n3034 = call <vilib>:"Write JPEG File.vi"("image data"=w3781, "path to JPEG file"=w3782) -> ()  [unwired: 8 in, 2 out]
                "Ref A Test Date :" <- "Ref A Test Date :"
                "Ref B Test Date :" <- "Ref B Test Date :"
                "Ref B Scar Value :" <- "Ref B Scar Value :"
                "Ref A Scar Value :" <- "Ref A Scar Value :"
              }
              frame #1 {
                (unwired) HTML_Report_Image_Alignment."MIDDLE" ("alignment (default)")
                w3818 = u16 0 items=["portrait", "landscape"] ("orientation (portrait)")
                (unwired) HTML_Report_Image_Alignment."ABSMIDDLE" ("alignment (default)")
                (unwired) "TESTED BY : "
                (unwired) "TESTED DATE :"
                (unwired) "SAMPLE ID : "
                (unwired) "SAMPLE DESIGN : "
                w3851 = "\r"
                # "add image"
                n3035 = Wait (ms)(milliseconds to wait=u32 20) -> ()  [unwired: 1 out]
                n3036 = local read "Sample ID  2"() -> (w3844:string)
                n3037 = local read "Wear Scar X"() -> (w3816:dbl)
                "Length ( microns ) 2" <- w3816
                n3038 = local read "Wear Scar Y"() -> (w3815:dbl)
                "Wear Scar Y ( microns ) :" <- w3815
                n3039 = local read "Test Date 2"() -> (w3845:string)
                n3040 = local read "Tested by 2"() -> (w3846:string)
                n3041 = local read "String 46"() -> (w3842:string)
                n3042 = local read "String 48"() -> (w3848:string)
                n3043 = local read "String 47"() -> (w3847:string)
                n3044 = local read "String 49"() -> (w3849:string)
                n3045 = local read "String 10"() -> (w3802:string)
                n3046 = local read "s.NO 2"() -> (w3843:string)
                n3047 = Add(x=w3816, y=w3815) -> (x+y=w3814:dbl)
                n3048 = call <vilib>:"New Report.vi"("report type"=enum16{"Standard Report", "HTML"}."HTML") -> ("report out"=w3822:refnum<class "NI_report.lvclass">, "error out"=w3820:errorcluster)  [unwired: 13 in]
                n3049 = Concatenate Strings(w3851, w3842, w3843, w3851, w3848, w3844, w3851, w3847, w3845, w3851, w3849, w3846, w3851) -> (→"test by 2":string)
                n3050 = Concatenate Strings("C:\\LAB-IQ\\Data\\" ("string"), w3802, ".jpg" ("string")) -> ()  [unwired: 1 out]
                n3051 = Divide(x=w3814, y=2.0) -> (x/y=→"Mean Wear ( microns) :":dbl)
                n3052 = call-dynamic "Set Report Orientation.vi"("report in"=w3822, "orientation (portrait)"=w3818, "error in (no error)"=w3820) -> ("report out"=w3821:refnum<class "NI_report.lvclass">, "error out"=w3819:errorcluster)  [unwired: 11 in]
                n3053 = for {
                  N: 5 -> [_]
                  tunnel: w3821 -> [w3872]
                  tunnel: [w3871] -> w3800
                  tunnel: w3819 -> [w3870]
                  tunnel: [w3869] -> w3799
                  n3054 = call-dynamic "Set Report Tab Width.vi"("report in"=w3872, "error in (no error)"=w3870) -> ("report out"=w3871:refnum<class "NI_report.lvclass">, "error out"=w3869:errorcluster)  [unwired: 12 in]
                }
                n3055 = local read "TITTLE"() -> (w3817:string)
                n3056 = call-dynamic "Set Report Header Text.vi"("report in"=w3800, "center header text"=w3817, "error in (no error)"=w3799) -> ("report out"=w3838:refnum<class "NI_report.lvclass">, "error out"=w3837:errorcluster)  [unwired: 11 in]
                n3057 = for {
                  N: 1 -> [_]
                  tunnel: [w3876] -> w3824
                  tunnel: [w3875] -> w3823
                  tunnel: w3838 -> [w3874]
                  tunnel: w3837 -> [w3873]
                  n3058 = call-dynamic "New Report Line.vi"("report in"=w3874, "error in (no error)"=w3873) -> ("report out"=w3876:refnum<class "NI_report.lvclass">, "error out"=w3875:errorcluster)  [unwired: 12 in]
                }
                n3059 = for {
                  N: 2 -> [_]
                  tunnel: [w3868] -> w3830
                  tunnel: [w3867] -> w3829
                  tunnel: w3824 -> [w3866]
                  tunnel: w3823 -> [w3865]
                  n3060 = call-dynamic "New Report Line.vi"("report in"=w3866, "error in (no error)"=w3865) -> ("report out"=w3868:refnum<class "NI_report.lvclass">, "error out"=w3867:errorcluster)  [unwired: 12 in]
                }
                n3061 = for {
                  N: 25 -> [_]
                  tunnel: w3830 -> [w3864]
                  tunnel: w3829 -> [w3862]
                  tunnel: [w3863] -> w3833
                  tunnel: [w3861] -> w3832
                  n3062 = call-dynamic "Set Report Tab Width.vi"("report in"=w3864, "error in (no error)"=w3862) -> ("report out"=w3863:refnum<class "NI_report.lvclass">, "error out"=w3861:errorcluster)  [unwired: 12 in]